vi "HFRR ADV v040.vi"() -> ()   [LabVIEW 2025] (continued)
                    n2687 = local read "FF 2"() -> (→"Frictional Force ( N )" →"Frictional Force ( N )":dbl)
                    n2688 = Build Path(base path=w3261, name or relative path=w3262) -> (appended path=w3257:path)
                    n2689 = flat-sequence {
                      tunnel: w3251 -> [w3317]
                      tunnel: [w3316] -> w3249
                      tunnel: w3248 -> [w3314]
                      tunnel: [w3319] -> w3250
                      tunnel: w3249 -> [w3319]
                      frame #0 {
                        n2690 = call <vilib>:"Mean PtByPt.vi"("x"=w3317, "sample length"="STROKE FILTER", "initialize"=w3314) -> ("mean"=w3316:dbl)  [unwired: 1 in, 1 out]
                      }
                      frame #1 {
                        "STROKE Initialize" <- FALSE ("STROKE Initialize")
                      }
                    }
                    n2691 = local read "COF 2"() -> (w3271:dbl)
                    "Coefficient of Friction" <- w3271
                    "COF 4" <- w3271
                    "Coefficient of Friction" <- w3271
                    n2692 = local read "TEMP"() -> (w3274:dbl)
                    "Temperature ( Deg C )" <- w3274
                    n2693 = local read "Humidity ( %RH )"() -> (w3273:dbl)
                    n2694 = local read "Frequency ( Hz )"() -> (w3280:dbl)
                    n2695 = local read "LVDT STROKE DISPLAY"() -> (w3252:dbl)
                    n2696 = local read "Elapsed time"() -> (w3305:dbl)
                    n2697 = local read "AIR TEMP"() -> (w3278:dbl)
                    n2698 = local read "PID-out"() -> (w3283:dbl)
                    n2699 = local write "Temperature ( Deg C )"(w3274) -> ()
                    n2700 = Number To Fractional String(number=w3252, width (-)=i16 9 ("precision (6)"), precision (6)=i16 6) -> (F-format string=w3298:string)  [unwired: 1 in]
                    n2701 = Number To Fractional String(number=w3278, width (-)=i16 9 ("precision (6)"), precision (6)=i16 3) -> (F-format string=w3297:string)  [unwired: 1 in]
                    n2702 = Number To Fractional String(number=w3274, width (-)=i16 9 ("precision (6)"), precision (6)=i16 3) -> (F-format string=w3294:string)  [unwired: 1 in]
                    n2703 = Number To Fractional String(number=w3273, width (-)=i16 9 ("precision (6)"), precision (6)=i16 3) -> (F-format string=w3291:string)  [unwired: 1 in]
                    n2704 = Number To Fractional String(number=0.0, width (-)=i16 9 ("precision (6)"), precision (6)=i16 3) -> (F-format string=w3288:string)  [unwired: 1 in]
                    n2705 = Number To Fractional String(number=w3283, width (-)=i16 9 ("precision (6)"), precision (6)=i16 3) -> (F-format string=w3284:string)  [unwired: 1 in]
                    n2706 = Number To Fractional String(number=w3280, width (-)=i16 9 ("precision (6)"), precision (6)=i16 3) -> (F-format string=w3279:string)  [unwired: 1 in]
                    n2707 = Number To Fractional String(number=w3271, width (-)=i16 9 ("precision (6)"), precision (6)=i16 6) -> (F-format string=w3306:string)  [unwired: 1 in]
                    n2708 = Number To Fractional String(number=w3305, width (-)=i16 14 ("precision (6)"), precision (6)=i16 3) -> (F-format string=w3307:string)  [unwired: 1 in]
                    n2709 = Bundle("y"=1.02, "LVDT STROKE DISPLAY"=w3252, "y"=0.98) -> (w3272:T31)  [unwired: 1 in]
                    n2710 = Number To Fractional String(number="Ambient Humidity :", width (-)=i16 9 ("precision (6)"), precision (6)=i16 6) -> (F-format string=w3264:string)  [unwired: 1 in]
                    n2711 = local read "RUN"() -> (w3270:bool)
                    n2712 = case shown="True" w3270 {
                      tunnel: w3272 -> [_ w3323]
                      tunnel: w3252 -> [_ w3322]
                      tunnel: w3252 -> [_ w3320]
                      tunnel: w3252 -> [_ w3321]
                      frame False {
                      }
                      frame True {
                        "Stroke ( mm )" <- w3323
                        "Stroke ( mm )" <- w3323
                        "Stroke 4" <- w3322
                        "Stroke 3" <- w3320
                        "Stroke 2" <- w3321
                        "measured_stroke" <- w3320
                      }
                    }
                    n2713 = Concatenate Strings(w3307, w3266, w3306, w3266, w3298, w3266, w3297, w3266, w3294, w3266, w3291, w3266, w3288, w3266, w3284, w3266, w3279, w3266, w3264, "\r") -> (w3304:string)
                    n2714 = call <vilib>:"Write Characters To File.vi"("append to file? (new file:F)"=TRUE, "character string"=w3304, "file path (dialog if empty)"=w3257) -> ()  [unwired: 2 in, 1 out]
                    "refresh flag" <- TRUE ("refresh flag")
                    "LVDT STROKE Actual" <- w3250
                  }
                }
                n2715 = case shown="True" w3172 {
                  tunnel: w3182 -> [_ w3208]
                  tunnel: w3187 -> [_ w3218]
                  tunnel: [0.0 w3214] -> _
                  tunnel: w3181 -> [_ w3213]
                  tunnel: [0.0 w3212] -> _
                  tunnel: w3171 -> [_ w3212]
                  tunnel: w3185 -> [w3201 _]
                  frame False {
                    n2716 = local write "acq timer"(w3201) -> ()
                    n2717 = local write "Test Duration Status"(0.0 ("Test Duration Status")) -> ()
                  }
                  frame True {
                    n2718 = local read "Set Hz"() -> (w3215:dbl)
                    n2719 = local write "Elapsed time"(w3208) -> ()
                    n2720 = local read "test time"() -> (w3207:dbl)
                    n2721 = Multiply(x=w3218, y=w3215) -> (x*y=w3217:dbl)
                    n2722 = case shown="False" w3213 {
                      tunnel: w3217 -> [w3219 _]
                      tunnel: [w3219 1.0] -> w3214
                      frame False {
                        n2723 = local write "Cycles elapsed"(w3219) -> ()
                      }
                      frame True {
                      }
                    }
                    n2724 = Greater?(x=w3208, y=w3207) -> (0:w3216:bool)
                    n2725 = Subtract(x=w3207, y=w3208) -> (x-y=w3206:dbl)
                    n2726 = Multiply(x=w3206, y=60.0) -> (x*y=w3205:dbl)
                    n2727 = local write "Time Remaining"(w3205) -> ()
                    n2728 = local write "Remaining Time"(w3205) -> ()
                    n2729 = case shown="True" w3216 {
                      frame False {
                      }
                      frame True {
                        n2730 = stacked-sequence {
                          frame #0 {
                            w3224 = T19."Enabled" ("Disabled")
                            w3223 = FALSE ("TEST FILE NAM,E SAVED")
                            w3225 = "" ("FILE")
                            w3226 = TRUE ("Visible")
                            n2731 = local write "Humidity"(FALSE ("Humidity")) -> ()
                            n2732 = local write "RUN"(FALSE ("OK Button 2")) -> ()
                            n2733 = local write "Heater Button"(FALSE ("Heater Button")) -> ()
                            n2734 = local write "Auto Start Test"(FALSE ("Auto Start Test")) -> ()
                            n2735 = local write "TestCompFlg"(TRUE ("StpFlg")) -> ()
                            n2736 = local read "Humidity ( %RH )"() -> (→"Rh After":dbl)
                            n2737 = property on="STOP 2" class="Bool (strict)"("Disabled"=u8 0) -> ()  [unwired: 2 in, 2 out]
                            n2738 = local read "EVENT LOG"() -> (w3231:string)
                            n2739 = call "Event Log.vi"("Content"="Test Completed", "EVENT LOG"=w3231) -> ("EVENT LOG"=w3230:string)  [unwired: 8 in, 1 out]
                            n2740 = property on="RUN" class="Bool (strict)"("Visible"=w3226) -> ()  [unwired: 2 in, 2 out]
                            n2741 = property on="Auto Start Test" class="Bool (strict)"("Visible"=w3226) -> ()  [unwired: 2 in, 2 out]
                            n2742 = local write "Batch Ref Num :"(w3225) -> ()
                            n2743 = local write "FILE"(w3225) -> ()
                            n2744 = local write "EVENT LOG"(w3230) -> ()
                            n2745 = local write "TEST FILE NAM,E SAVED"(w3223) -> ()
                            n2746 = local write "Fuel Discription :"(w3225) -> ()
                            n2747 = local write "START TEMP"(w3223) -> ()
                            n2748 = local write "Remarks :"(w3225) -> ()
                            n2749 = local write "Main Dashboard Buttons"(T1."Imaging" ("Main Dashboard Buttons")) -> ()
                            n2750 = local write "Main Tab"(T2."Adv Scar" ("Main Tab")) -> ()
                            n2751 = property on="FRICVALZ 2" class="Bool (strict)"("DisabledEnum"=w3224) -> ()  [unwired: 2 in, 2 out]
                            n2752 = property on="FRICVALZ 3" class="Bool (strict)"("DisabledEnum"=w3224) -> ()  [unwired: 2 in, 2 out]
                            n2753 = property on="FRICVALZ 4" class="Bool (strict)"("DisabledEnum"=w3224) -> ()  [unwired: 2 in, 2 out]
                          }
                          frame #1 {
                            n2754 = Wait (ms)(milliseconds to wait=u32 1500) -> ()  [unwired: 1 out]
                          }
                          frame #2 {
                            n2755 = local write "Due Write"("VC;0") -> ()
                          }
                          frame #3 {
                            n2756 = Wait (ms)(milliseconds to wait=u32 1500) -> ()  [unwired: 1 out]
                          }
                          frame #4 {
                            n2757 = local write "Due Write"("VC;0") -> ()
                          }
                          frame #5 {
                            n2758 = Wait (ms)(milliseconds to wait=u32 1500) -> ()  [unwired: 1 out]
                          }
                          frame #6 {
                            n2759 = local write "Due Write"("ST;0") -> ()
                          }
                          frame #7 {
                            n2760 = local write "measured_stroke"(0.0 ("measured_stroke")) -> ()
                            n2761 = Wait (ms)(milliseconds to wait=u32 1500) -> ()  [unwired: 1 out]
                          }
                          frame #8 {
                            n2762 = local write "Due Write"("HE;0") -> ()
                            n2763 = local write "Humidity 2"(TRUE ("Humidity")) -> ()
                          }
                        }
                      }
                    }
                    n2764 = Divide(x=w3208, y=w3207) -> (x/y=w3211:dbl)
                    n2765 = Multiply(x=w3211, y=100.0) -> (x*y=w3209:dbl)
                    n2766 = local write "Test Duration Status"(w3209) -> ()
                  }
                }
              }
              frame #2 {
                n2767 = case shown="True" "Heater Button" {
                  tunnel: [0.0 ("output") w3346] -> w3324
                  frame False {
                    w3327 = TRUE ("tmpchk")
                    n2768 = local read "TEMP"() -> (w3328:dbl)
                    n2769 = local write "Temp ini"(w3328) -> ()
                    n2770 = local write "Reset 4"(w3327) -> ()
                    n2771 = local write "tmpchk"(w3327) -> ()
                    n2772 = local write "reinit"(TRUE ("reinit")) -> ()
                    n2773 = local write "manual temp log"(TRUE ("manual temp log")) -> ()
                  }
                  frame True {
                    # "Logic to turn off\nthe heater when \ntemp is not rising.\nTime - 60 sec\nDelta t- 5°c"
                    n2774 = local read "Temp ini"() -> (w3335:dbl)
                    n2775 = local read "Auto Start Test"() -> (w3331:bool)
                    n2776 = Less?(x=w3335, y=53.0) -> (x < y?=w3333:bool)
                    n2777 = case shown="False" w3331 {
                      frame False {
                        n2778 = local read "Set Temp"() -> (w3355:dbl)
                        n2779 = local read "TEMP"() -> (w3354:dbl)
                        n2780 = Subtract(x=w3355, y=w3354) -> (x-y=w3353:dbl)
                        n2781 = Absolute Value(x=w3353) -> (abs(x)=w3352:dbl)
                        n2782 = Less?(x=w3352, y=0.5) -> (x < y?=w3350:bool)
                        n2783 = case shown="True" w3350 {
                          tunnel: "manual temp log" -> [_ w3356]
                          frame False {
                          }
                          frame True {
                            n2784 = case shown="True" w3356 {
                              selector: w3356 -> [_ w3357]
                              frame False {
                              }
                              frame True {
                                # "#Event log"
                                n2785 = Not(x=w3357) -> (.not. x?=w3358:bool)
                                n2786 = local write "manual temp log"(w3358) -> ()
                                n2787 = local read "EVENT LOG"() -> (w3361:string)
                                n2788 = call "Event Log.vi"("Content"="Target Temperature reached", "EVENT LOG"=w3361) -> ("EVENT LOG"=w3360:string)  [unwired: 8 in, 1 out]
                                n2789 = local write "EVENT LOG"(w3360) -> ()
                              }
                            }
                          }
                        }
                      }
                      frame True {
                        n2790 = local write "manual temp log"(TRUE ("manual temp log")) -> ()
                      }
                    }
                    n2791 = And(x="tmpchk", y=w3333) -> (x .and. y?=w3336:bool)
                    n2792 = case shown="True" w3336 {
                      frame False {
                      }
                      frame True {
                        n2793 = call "Elapsed Time8"("Time Target (s)"=300.0, "Reset"="Reset 4") -> ("Time has Elapsed"=w3363:bool)  [unwired: 10 in, 7 out]
                        n2794 = flat-sequence {
                          tunnel: w3363 -> [_]
                          frame #0 {
                            n2795 = local write "Reset 4"(FALSE ("Reset 4")) -> ()
                          }
                        }
                        n2796 = case shown="True" w3363 {
                          frame False {
                          }
                          frame True {
                            n2797 = local read "Temp ini"() -> (w3370:dbl)
                            n2798 = Add(x=w3370, y=5.0) -> (x+y=w3368:dbl)
                            n2799 = local read "TEMP"() -> (w3371:dbl)
                            n2800 = Greater?(x=w3371, y=w3368) -> (0:w3369:bool)
                            n2801 = case shown="False" w3369 {
                              frame False {
                                n2802 = local write "Heater Button"(FALSE ("Heater Button")) -> ()
                              }
                              frame True {
                                n2803 = local write "tmpchk"(FALSE ("tmpchk")) -> ()
                              }
                            }
                          }
                        }
                      }
                    }
                    n2804 = local read "Set Temp"() -> (w3344:dbl)
                    n2805 = local read "TEMP"() -> (w3338:dbl)
                    n2806 = call-poly <vilib>:"PID.vi"("reinitialize? (F)"="reinit", "dt (s)"=-1.0, "process variable"=w3338, "setpoint"=w3344) -> ("output"=w3341:dbl)  [unwired: 6 in, 1 out]
                    n2807 = Subtract(x=w3344, y=w3338) -> (x-y=w3345:dbl)
                    n2808 = Add(x=w3344, y=0.5) -> (x+y=w3342:dbl)
                    n2809 = Greater Or Equal?(x=w3338, y=w3342) -> ()  [unwired: 1 out]
                    n2810 = Select(t=0.0, s=FALSE, f=w3341) -> (s? t:f=w3340:dbl)
                    "PID output" <- w3340
                    n2811 = flat-sequence {
                      tunnel: w3340 -> [w3374]
                      tunnel: [w3374] -> w3346
                      frame #0 {
                        n2812 = local write "reinit"(FALSE ("reinit")) -> ()
                      }
                    }
                    n2813 = Bundle(w3345, "output"=w3340, "TEMP"=w3338) -> ()  [unwired: 1 in, 1 out]
                  }
                }
                "PID-out" <- w3324
              }
              frame #3 {
                n2814 = local read "TEMP"() -> (w3376:dbl)
                n2815 = Greater Or Equal?(x=w3376, y="Set Temp 2") -> (x >= y?=w3381:bool)
                n2816 = case shown="True" w3381 {
                  tunnel: [FALSE TRUE] -> w3379
                  frame False {
                  }
                  frame True {
                  }
                }
                "Status 13" <- w3379
                n2817 = And(x=w3379, y="trip1 8") -> (x .and. y?=w3378:bool)
                n2818 = case shown="True" w3378 {
                  frame False {
                    n2819 = local write "Heater Trip Temp"(TRUE ("Heater Trip Temp")) -> ()
                  }
                  frame True {
                    w3384 = FALSE ("OK Button 2")
                    n2820 = case shown="True" "Heater Trip Temp" {
                      selector: "Heater Trip Temp" -> [_ w3386]
                      frame False {
                      }
                      frame True {
                        n2821 = Not(x=w3386) -> (.not. x?=w3385:bool)
                        n2822 = local read "EVENT LOG"() -> (w3389:string)
                        n2823 = local write "Heater Trip Temp"(w3385) -> ()
                        n2824 = call "Event Log.vi"("Content"="Heater Trip", "EVENT LOG"=w3389) -> ("EVENT LOG"=w3388:string)  [unwired: 8 in, 1 out]
                        n2825 = local write "EVENT LOG"(w3388) -> ()
                      }
                    }
                    n2826 = local write "RUN"(w3384) -> ()
                    n2827 = property on="Auto Start Test" class="Bool (strict)"("Value"=w3384) -> ()  [unwired: 2 in, 2 out]
                    n2828 = local write "Heater Button"(w3384) -> ()
                  }
                }
              }
            }
            n2829 = case shown="False" w3095 {
              frame False {
                n2830 = disable-structure shown="Disabled" {
                  frame Disabled {
                    n2831 = stacked-sequence {
                      frame #0 {
                        n2832 = local write "RUN"(FALSE ("OK Button 2")) -> ()
                      }
                      frame #1 {
                      }
                    }
                  }
                  frame Enabled {
                  }
                }
              }
              frame True {
              }
            }
          }
        }
        n2833 = local read "Reset Graph"() -> (w2992:bool)
        n2834 = case shown="True" w2992 {
          selector: w2992 -> [_ w3009]
          frame False {
          }
          frame True {
            w3023 = 0.0 ("X Scale.Range:Maximum")
            n2835 = Not(x=w3009) -> (.not. x?=w3008:bool)
            n2836 = local write "Reset Graph"(w3008) -> ()
            n2837 = property on="Electrical Contact Resistance ( % )" class="WFChart (strict)"("XScale.Maximum"=600.0 ("X Scale.Range:Maximum"), "XScale.Minimum"=0.0 ("X Scale.Range:Minimum"), "YScale.Maximum"=100.0 ("Y Scale.Range:Maximum"), "YScale.Minimum"=0.0 ("Y Scale.Range:Minimum")) -> ()  [unwired: 2 in, 2 out]
            n2838 = property on="Frictional Force ( N )" class="WFChart (strict)"("XScale.Maximum"=600.0 ("X Scale.Range:Maximum"), "XScale.Minimum"=0.0 ("X Scale.Range:Minimum"), "YScale.Maximum"=100.0 ("Y Scale.Range:Maximum"), "YScale.Minimum"=0.0 ("Y Scale.Range:Minimum")) -> ()  [unwired: 2 in, 2 out]
            n2839 = property on="Temperature ( Deg C )" class="WFChart (strict)"("XScale.Maximum"=600.0 ("X Scale.Range:Maximum"), "XScale.Minimum"=0.0 ("X Scale.Range:Minimum"), "YScale.Maximum"=100.0 ("Y Scale.Range:Maximum"), "YScale.Minimum"=0.0 ("Y Scale.Range:Minimum")) -> ()  [unwired: 2 in, 2 out]
            n2840 = property on="Stroke ( mm )" class="WFChart (strict)"("XScale.Maximum"=600.0 ("X Scale.Range:Maximum"), "XScale.Minimum"=0.0 ("X Scale.Range:Minimum"), "YScale.Maximum"=100.0 ("Y Scale.Range:Maximum"), "YScale.Minimum"=0.0 ("Y Scale.Range:Minimum")) -> ()  [unwired: 2 in, 2 out]
            n2841 = property on="Coefficient of Friction" class="WFChart (strict)"("XScale.Maximum"=600.0 ("X Scale.Range:Maximum"), "XScale.Minimum"=0.0 ("X Scale.Range:Minimum"), "YScale.Maximum"=100.0 ("Y Scale.Range:Maximum"), "YScale.Minimum"=0.0 ("Y Scale.Range:Minimum")) -> ()  [unwired: 2 in, 2 out]
            n2842 = property on="Electrical Contact Resistance ( % )" class="WFChart (strict)"("XScale.Minimum"=0.0 ("X Scale.Range:Minimum"), "XScale.Maximum"=600.0 ("X Scale.Range:Maximum"), "YScale.Minimum"=0.0 ("Y Scale.Range:Minimum"), "YScale.Maximum"=100.0 ("Y Scale.Range:Maximum")) -> ()  [unwired: 2 in, 2 out]
            n2843 = property on="Temperature ( Deg C )" class="WFChart (strict)"("XScale.Minimum"=0.0 ("X Scale.Range:Minimum"), "XScale.Maximum"=600.0 ("X Scale.Range:Maximum"), "YScale.Minimum"=0.0 ("Y Scale.Range:Minimum"), "YScale.Maximum"=100.0 ("Y Scale.Range:Maximum")) -> ()  [unwired: 2 in, 2 out]
            n2844 = property on="Coefficient of Friction" class="WFChart (strict)"("XScale.Minimum"=0.0 ("X Scale.Range:Minimum"), "XScale.Maximum"=600.0 ("X Scale.Range:Maximum"), "YScale.Maximum"=1.0 ("X Scale.Range:Minimum"), "YScale.Minimum"=0.0 ("X Scale.Range:Minimum")) -> ()  [unwired: 2 in, 2 out]
            n2845 = property on="Frictional Force ( N )" class="WFChart (strict)"("XScale.Maximum"=600.0 ("X Scale.Range:Maximum"), "XScale.Minimum"=w3023, "YScale.Maximum"=10.0 ("Y Scale.Range:Maximum"), "YScale.Minimum"=w3023) -> ()  [unwired: 2 in, 2 out]
            n2846 = property on="Stroke ( mm )" class="WFChart (strict)"("XScale.Maximum"=600.0 ("X Scale.Range:Maximum"), "XScale.Minimum"=0.0 ("X Scale.Range:Minimum"), "YScale.Maximum"=100.0 ("Y Scale.Range:Maximum"), "YScale.Minimum"=0.0 ("Y Scale.Range:Minimum")) -> ()  [unwired: 2 in, 2 out]
          }
        }
      }
      frame "Compare Files" {
        # "Elapsed time\ncof\nstroke\nAir temp\nTemp\nHumidity"
        n2847 = case shown="True" "RSTV1 2" {
          frame False {
          }
          frame True {
            n2848 = property on="Humidity ( %RH )" class="XYGraph (strict)"("Y Scale.Display Format:Precision"=u8 0 ("Y Scale.Format & Precision:Precision")) -> ()  [unwired: 2 in, 2 out]
            n2849 = property on="Humidity ( %RH )" class="XYGraph (strict)"("X Scale.Range:Minimum"=0.0, "X Scale.Range:Maximum"=75.0, "Y Scale.Range:Minimum"=48.0, "Y Scale.Range:Maximum"=58.0) -> ()  [unwired: 2 in, 2 out]
          }
        }
        n2850 = case shown="True" "RST CP 2" {
          frame False {
          }
          frame True {
            n2851 = property on="XY Graph 13" class="XYGraph (strict)"("Y Scale.Display Format:Precision"=u8 0 ("Y Scale.Format & Precision:Precision")) -> ()  [unwired: 2 in, 2 out]
            n2852 = property on="XY Graph 13" class="XYGraph (strict)"("X Scale.Range:Minimum"=0.0, "X Scale.Range:Maximum"=75.0, "Y Scale.Range:Minimum"=0.0, "Y Scale.Range:Maximum"=100.0) -> ()  [unwired: 2 in, 2 out]
          }
        }
        n2853 = case shown="True" "RST CP" {
          frame False {
          }
          frame True {
            n2854 = property on="Sample Temperature ( °C )" class="XYGraph (strict)"("Y Scale.Display Format:Precision"=u8 2 ("Y Scale.Format & Precision:Precision")) -> ()  [unwired: 2 in, 2 out]
            n2855 = property on="Sample Temperature ( °C )" class="XYGraph (strict)"("X Scale.Range:Minimum"=0.0, "X Scale.Range:Maximum"=75.0, "Y Scale.Range:Minimum"=58.0, "Y Scale.Range:Maximum"=62.0) -> ()  [unwired: 2 in, 2 out]
          }
        }
        n2856 = case shown="True" "RSTV1 3" {
          frame False {
          }
          frame True {
            n2857 = property on="Air Temperature  ( °C )" class="XYGraph (strict)"("Y Scale.Display Format:Precision"=u8 2 ("Y Scale.Format & Precision:Precision")) -> ()  [unwired: 2 in, 2 out]
            n2858 = property on="Air Temperature  ( °C )" class="XYGraph (strict)"("X Scale.Range:Minimum"=0.0 ("Y Scale.Range:Minimum"), "X Scale.Range:Maximum"=75.0 ("Y Scale.Range:Maximum"), "Y Scale.Range:Minimum"=20.0 ("X Scale.Range:Minimum"), "Y Scale.Range:Maximum"=26.0 ("X Scale.Range:Maximum")) -> ()  [unwired: 2 in, 2 out]
          }
        }
        n2859 = case shown="True" "RSTV1 4" {
          frame False {
          }
          frame True {
            n2860 = property on="Stroke ( mm )" class="XYGraph (strict)"("Y Scale.Display Format:Precision"=u8 2 ("Y Scale.Format & Precision:Precision")) -> ()  [unwired: 2 in, 2 out]
            n2861 = property on="Stroke ( mm )" class="XYGraph (strict)"("X Scale.Range:Minimum"=0.0 ("Y Scale.Range:Maximum"), "X Scale.Range:Maximum"=75.0 ("X Scale.Range:Minimum"), "Y Scale.Range:Minimum"=0.98, "Y Scale.Range:Maximum"=1.02) -> ()  [unwired: 2 in, 2 out]
          }
        }
        n2862 = case shown="True" "rstv2" {
          frame False {
          }
          frame True {
            n2863 = property on="Coefficient Of Friction" class="XYGraph (strict)"("Y Scale.Display Format:Precision"=u8 3 ("Y Scale.Format & Precision:Precision")) -> ()  [unwired: 2 in, 2 out]
            n2864 = property on="Coefficient Of Friction" class="XYGraph (strict)"("X Scale.Range:Minimum"=0.0 ("Y Scale.Range:Maximum"), "X Scale.Range:Maximum"=75.0, "Y Scale.Range:Minimum"=0.0, "Y Scale.Range:Maximum"=1.0 ("X Scale.Range:Minimum")) -> ()  [unwired: 2 in, 2 out]
          }
        }
        n2865 = case shown="True" "RST CP 3" {
          frame False {
          }
          frame True {
            n2866 = property on="Air Temp ( °C ) vs Humidity ( % RH )" class="XYGraph (strict)"("X Scale.Range:Minimum"=18.0, "X Scale.Range:Maximum"=28.0 ("X Scale.Range:Minimum"), "Y Scale.Range:Minimum"=30.0 ("X Scale.Range:Minimum"), "Y Scale.Range:Maximum"=70.0 ("X Scale.Range:Minimum")) -> ()  [unwired: 2 in, 2 out]
          }
        }
        n2867 = case shown="True" "OPEN 1" {
          frame False {
          }
          frame True {
            (unwired) 0  # existing file
            w3665 = "Choose a datalog file to open"  # prompt
            n2868 = local write "OPEN 1"(FALSE ("OPEN 1")) -> ()
            n2869 = String To Path(string="C:\\LAB-IQ\\Data\\") -> (path=w3650:path)
            n2870 = File Dialog(6:"*.dgf" ("pattern"), 7:w3665, 11:w3650) -> (0:w3648:errorcluster, 3:w3656:path)  [unwired: 4 in, 2 out]
            n2871 = Unbundle(w3648) -> ()  [unwired: 3 out]
            n2872 = Strip Path(path=w3656) -> (name=w3655:string)  [unwired: 1 out]
            n2873 = Path To String(path=w3656) -> (string=w3651:string)
            "string1" <- w3651
            n2874 = Match Pattern(string=w3655, regular expression=".dgf") -> (before substring=→"String Control":string)  [unwired: 1 in, 3 out]
            n2875 = Match Pattern(string=w3651, regular expression=".dgf" ("substring (\"\")")) -> (before substring=w3661:string)  [unwired: 1 in, 3 out]
            n2876 = Concatenate Strings(w3661, ".duf" ("Substring")) -> (w3657:string)
            n2877 = String To Path(string=w3657) -> (path=w3662:path)
            n2878 = call <vilib>:"Read Characters From File.vi"("file path (dialog if empty)"=w3662, "start of read offset (chars.:0)"=60 ("start of read offset (chars.: 0)")) -> ("character string"=→"String Control 2":string)  [unwired: 4 in, 3 out]
          }
        }
        n2879 = case shown="True" "OPEN 2" {
          frame False {
          }
          frame True {
            (unwired) 0  # existing file
            w3683 = "Choose a datalog file to open"  # prompt
            n2880 = local write "OPEN 2"(FALSE ("OPEN 1")) -> ()
            n2881 = String To Path(string="C:\\LAB-IQ\\Data\\") -> (path=w3668:path)
            n2882 = File Dialog(6:"*.dgf" ("pattern"), 7:w3683, 11:w3668) -> (0:w3666:errorcluster, 3:w3674:path)  [unwired: 4 in, 2 out]
            n2883 = Unbundle(w3666) -> ()  [unwired: 3 out]
            n2884 = Strip Path(path=w3674) -> (name=w3672:string)  [unwired: 1 out]
            n2885 = Path To String(path=w3674) -> (string=w3669:string)
            "string1 2" <- w3669
            n2886 = Match Pattern(string=w3672, regular expression=".dgf") -> (before substring=→"String Control 3":string)  [unwired: 1 in, 3 out]
            n2887 = Match Pattern(string=w3669, regular expression=".dgf" ("substring (\"\")")) -> (before substring=w3680:string)  [unwired: 1 in, 3 out]
            n2888 = Concatenate Strings(w3680, ".duf" ("Substring")) -> (w3677:string)
            n2889 = String To Path(string=w3677) -> (path=w3675:path)
            n2890 = call <vilib>:"Read Characters From File.vi"("file path (dialog if empty)"=w3675, "start of read offset (chars.:0)"=60 ("start of read offset (chars.: 0)")) -> ("character string"=→"String Control 4":string)  [unwired: 4 in, 3 out]
          }
        }
        n2891 = case shown="True" "OPEN 3" {
          frame False {
          }
          frame True {
            (unwired) 0  # existing file
            w3701 = "Choose a datalog file to open"  # prompt
            n2892 = local write "OPEN 3"(FALSE ("OPEN 1")) -> ()
            n2893 = String To Path(string="C:\\LAB-IQ\\Data\\") -> (path=w3686:path)
            n2894 = File Dialog(6:"*.dgf" ("pattern"), 7:w3701, 11:w3686) -> (0:w3684:errorcluster, 3:w3692:path)  [unwired: 4 in, 2 out]
            n2895 = Unbundle(w3684) -> ()  [unwired: 3 out]
            n2896 = Strip Path(path=w3692) -> (name=w3690:string)  [unwired: 1 out]
            n2897 = Path To String(path=w3692) -> (string=w3687:string)
            "string1 3" <- w3687
            n2898 = Match Pattern(string=w3690, regular expression=".dgf") -> (before substring=→"String Control 5":string)  [unwired: 1 in, 3 out]
            n2899 = Match Pattern(string=w3687, regular expression=".dgf" ("substring (\"\")")) -> (before substring=w3697:string)  [unwired: 1 in, 3 out]
            n2900 = Concatenate Strings(w3697, ".duf" ("Substring")) -> (w3694:string)
            n2901 = String To Path(string=w3694) -> (path=w3698:path)
            n2902 = call <vilib>:"Read Characters From File.vi"("file path (dialog if empty)"=w3698, "start of read offset (chars.:0)"=60 ("start of read offset (chars.: 0)")) -> ("character string"=→"String Control 6":string)  [unwired: 4 in, 3 out]
          }
        }
        n2903 = case shown="True" "OPEN 4" {
          frame False {
          }
          frame True {
            (unwired) 0  # existing file
            w3719 = "Choose a datalog file to open"  # prompt
            n2904 = local write "OPEN 4"(FALSE ("OPEN 1")) -> ()
            n2905 = String To Path(string="C:\\LAB-IQ\\Data\\") -> (path=w3704:path)
            n2906 = File Dialog(6:"*.dgf" ("pattern"), 7:w3719, 11:w3704) -> (0:w3702:errorcluster, 3:w3710:path)  [unwired: 4 in, 2 out]
            n2907 = Unbundle(w3702) -> ()  [unwired: 3 out]
            n2908 = Strip Path(path=w3710) -> (name=w3708:string)  [unwired: 1 out]
            n2909 = Path To String(path=w3710) -> (string=w3705:string)
            "string1 4" <- w3705
            n2910 = Match Pattern(string=w3708, regular expression=".dgf") -> (before substring=→"String Control 7":string)  [unwired: 1 in, 3 out]
            n2911 = Match Pattern(string=w3705, regular expression=".dgf" ("substring (\"\")")) -> (before substring=w3715:string)  [unwired: 1 in, 3 out]
            n2912 = Concatenate Strings(w3715, ".duf" ("Substring")) -> (w3712:string)
            n2913 = String To Path(string=w3712) -> (path=w3716:path)
            n2914 = call <vilib>:"Read Characters From File.vi"("file path (dialog if empty)"=w3716, "start of read offset (chars.:0)"=60 ("start of read offset (chars.: 0)")) -> ("character string"=→"String Control 8":string)  [unwired: 4 in, 3 out]
          }
        }
      }
      frame "About" {
        # "Elapsed time\ncof\nstroke\nmean pos\nTemp\nHumidity"
        n2915 = disable-structure shown="Disabled" {
          frame Disabled {
            n2916 = case shown="True" "Export" {
              frame False {
              }
              frame True {
                w3741 = "                                      " ("string")
                w3743 = "\r"
                (unwired) i16 6 ("width (-)")
                w3820 = "\r"
                w3752 = "\r"
                n2917 = local write "Export"(FALSE ("Export")) -> ()
                n2918 = local read "String 29"() -> (w3789:string)
                n2919 = local read "String 34"() -> (w3777:string)
                n2920 = local read "String 35"() -> (w3772:string)
                n2921 = local read "String 37"() -> (w3768:string)
                n2922 = local read "String 36"() -> (w3765:string)
                n2923 = local read "String 38"() -> (w3762:string)
                n2924 = local read "String 39"() -> (w3759:string)
                n2925 = Match Pattern(string=w3789, regular expression=".dwm") -> (before substring=w3785:string)  [unwired: 1 in, 3 out]
                "before substring" <- w3785
                n2926 = local read "S 38"() -> (w3780:string)
                n2927 = local read "S 39"() -> (w3773:string)
                n2928 = local read "Temperature before test 2"() -> (w3809:dbl)
                n2929 = local read "Temperature after test 2"() -> (w3814:dbl)
                n2930 = local read "Humidity before test 2"() -> (w3795:dbl)
                n2931 = local read "Humidity after test 2"() -> (w3810:dbl)
                n2932 = local read "MWSD 2"() -> (w3806:dbl)
                n2933 = local read "WS1.4 2"() -> (w3822:dbl)
                n2934 = local read "HCF 2"() -> (w3818:dbl)
                n2935 = local read "AVP 2"() -> (w3807:dbl)
                n2936 = Concatenate Strings("1," ("string"), w3780) -> (w3779:string)
                n2937 = Concatenate Strings("2," ("string"), w3777) -> (w3776:string)
                n2938 = Concatenate Strings("3," ("string"), w3773) -> (w3775:string)
                n2939 = Concatenate Strings("4," ("string"), w3772) -> (w3771:string)
                n2940 = Concatenate Strings("5," ("string"), w3768) -> (w3769:string)
                n2941 = Concatenate Strings("6," ("string"), w3765) -> (w3766:string)
                n2942 = Concatenate Strings("7," ("string"), w3762) -> (w3763:string)
                n2943 = Concatenate Strings("8," ("string"), w3759) -> (w3760:string)
                n2944 = local read "Sample ID"() -> (w3827:string)
                n2945 = case shown="\"xlx\"" "Select File Type" {
                  tunnel: w3785 -> [w3830 w3832 w3834]
                  tunnel: [w3828 w3833 w3835] -> w3784
                  frame "xlx" {
                    n2946 = Concatenate Strings(w3830, ".xls" ("string")) -> (w3828:string)
                  }
                  frame "csv" {
                    n2947 = Concatenate Strings(w3832, ".csv" ("string")) -> (w3833:string)
                  }
                  frame "txt" {
                    n2948 = Concatenate Strings(w3834, ".txt" ("string")) -> (w3835:string)
                  }
                }
                n2949 = local read "Test Date"() -> (w3826:string)
                n2950 = local read "String 45"() -> (w3740:string)
                n2951 = local read "String 31"() -> (w3825:string)
                n2952 = local read "String 32"() -> (w3824:string)
                n2953 = local read "TITTLE"() -> (w3748:string)
                n2954 = Number To Fractional String(number=w3795, width (-)=i16 6, precision (6)=i16 2) -> (F-format string=w3794:string)  [unwired: 1 in]
                n2955 = Number To Fractional String(number=w3809, width (-)=i16 6, precision (6)=i16 2) -> (F-format string=w3815:string)  [unwired: 1 in]
                n2956 = Number To Fractional String(number=w3810, width (-)=i16 6, precision (6)=i16 2) -> (F-format string=w3808:string)  [unwired: 1 in]
                n2957 = Number To Fractional String(number=w3814, width (-)=i16 6, precision (6)=i16 2) -> (F-format string=w3813:string)  [unwired: 1 in]
                n2958 = Number To Fractional String(number=w3806, width (-)=i16 6, precision (6)=i16 2) -> (F-format string=w3804:string)  [unwired: 1 in]
                n2959 = Number To Fractional String(number=w3807, width (-)=i16 6, precision (6)=i16 2) -> (F-format string=w3805:string)  [unwired: 1 in]
                n2960 = Number To Fractional String(number=w3818, width (-)=i16 6, precision (6)=i16 2) -> (F-format string=w3819:string)  [unwired: 1 in]
                n2961 = Number To Fractional String(number=w3822, precision (6)=i16 2) -> (F-format string=w3823:string)  [unwired: 2 in]
                n2962 = local read "s.NO"() -> (w3742:string)
                n2963 = Concatenate Strings("=" ("string"), w3748) -> (w3747:string)
                n2964 = Concatenate Strings("S.No," ("string"), "                                       Parameters" ("string")) -> (w3753:string)
                n2965 = Concatenate Strings(w3820, w3779, w3794, w3820, w3776, w3815, w3820, w3775, w3808, w3820, w3771, w3813, w3820, w3769, w3804, w3820, w3766, w3805, w3820, w3763, w3819, w3820, w3760, w3823) -> (w3782:string)
                n2966 = Concatenate Strings(w3752, "," ("string"), w3740, w3742, w3741, w3824, w3827, w3741, w3825, w3826, w3752) -> (w3750:string)
                n2967 = local read "Tested by"() -> (w3756:string)
                n2968 = local read "String 33"() -> (w3757:string)
                n2969 = Concatenate Strings("," ("string"), "                                                                             " ("string")) -> (w3745:string)
                n2970 = Concatenate Strings(w3747, w3743, w3750, w3743, w3753, w3782, w3743, w3745, w3757, w3756) -> (→"export":string)
                n2971 = String To Path(string=w3784) -> (path=w3791:path)
                n2972 = local read "export"() -> (w3786:string)
                n2973 = call <vilib>:"Write Characters To File.vi"("append to file? (new file:F)"=FALSE, "character string"=w3786, "file path (dialog if empty)"=w3791) -> ()  [unwired: 2 in, 1 out]
              }
            }
          }
          frame Enabled {
          }
        }
        n2974 = case shown="True" "OK Button 17" {
          frame False {
          }
          frame True {
            (unwired) 0  # existing file
            w4044 = "Choose a datalog file to open"  # prompt
            n2975 = local write "OK Button 17"(FALSE ("OK Button 17")) -> ()
            n2976 = local read "String"() -> (w4039:string)
            n2977 = String To Path(string=w4039) -> (path=w4040:path)
            n2978 = File Dialog(6:"*.duf" ("pattern"), 7:w4044, 11:w4040) -> (0:w4031:errorcluster, 3:w4050:path)  [unwired: 4 in, 2 out]
            n2979 = Unbundle(w4031) -> ()  [unwired: 3 out]
            n2980 = Open/Create/Replace File "Open File"(file path (use dialog)=w4050) -> (refnum out=w4042:refnum<file>)  [unwired: 5 in, 2 out]
            n2981 = Strip Path(path=w4050) -> (name=w4048:string)  [unwired: 1 out]
            n2982 = Path To String(path=w4050) -> (string=w4033:string)
            n2983 = while {
              tunnel: w4042 -> [w4054]
              i -> [w4051]
              stop <- w4052 continue-if-true
              (unwired) TRUE ("line mode (F)")
              n2984 = Read from Text File "Read File"(file (use dialog)=w4054) -> (text=w4053:string)  [unwired: 3 in, 3 out]
              n2985 = local write "Numeric 16"(w4051) -> ()
              n2986 = String Length(string=w4053) -> (length=w4056:i32)
              n2987 = Greater?(x=w4056, y=1) -> (0:w4052:bool)
            }
            n2988 = local write "String 29"(w4033) -> ()
            n2989 = Search and Replace String(input string=w4033, search string=".duf", replace string=".dgf" ("replace string (\"\")")) -> (result string=→"String Indicator 4":string)  [unwired: 5 in, 3 out]
            n2990 = Match Pattern(string=w4048, regular expression=".dwm") -> (before substring=w4032:string)  [unwired: 1 in, 3 out]
            "String Indicator" <- w4032
            n2991 = Match Pattern(string=w4033, regular expression=".dwm" ("substring (\"\")")) -> (before substring=w4034:string)  [unwired: 1 in, 3 out]
            "String Indicator 3" <- w4034
            n2992 = local write "TITTLE 2"(w4032) -> ()
            n2993 = String To Path(string=w4034) -> (path=w4041:path)
            "path" <- w4041
            n2994 = call <vilib>:"Read Characters From File.vi"("file path (dialog if empty)"=w4041, "start of read offset (chars.:0)"=60 ("start of read offset (chars.: 0)")) -> ("character string"=→"String Indicator 2":string)  [unwired: 4 in, 3 out]
          }
        }
        n2995 = call <vilib>:"Query Available Printers.vi"() -> ("system configured printers"=w3733:string[])  [unwired: 9 in, 2 out]
        "System Configured Printers 2" <- w3733
        n2996 = local read "OK Button 16"() -> (w3730:bool)
        n2997 = case shown="True" "OK Button 16" {
          frame False {
          }
          frame True {
            n2998 = stacked-sequence {
              frame #0 {
                n2999 = local read "Numeric 16"() -> (w4058:i32)
                n3000 = local write "Numeric 10"(w4058) -> ()
              }
              frame #1 {
                n3001 = local read "String 29"() -> (w4061:string)
                n3002 = String To Path(string=w4061) -> (path=w4060:path)
                n3003 = Open/Create/Replace File "Open File"(file path (use dialog)=w4060) -> (refnum out=w4062:refnum<file>)  [unwired: 5 in, 2 out]
                n3004 = for {
                  N: 16 -> [_]
                  tunnel: w4062 -> [w4069]
                  i -> [w4065]
                  (unwired) TRUE ("line mode (F)")
                  n3005 = Read from Text File "Read File"(file (use dialog)=w4069) -> (text=w4063:string)  [unwired: 3 in, 3 out]
                  n3006 = Match Pattern(string=w4063, regular expression="(") -> (after substring=w4068:string)  [unwired: 1 in, 3 out]
                  n3007 = Match Pattern(string=w4068, regular expression=")") -> (before substring=w4064:string)  [unwired: 1 in, 3 out]
                  n3008 = case shown="1" w4065 {
                    tunnel: w4064 -> [w4070 w4071 _ _ w4072 w4073 w4074 w4076 w4078 w4080 w4082 w4084 w4086 w4088 _]
                    tunnel: w4063 -> [_ _ _ _ _ _ _ _ _ _ _ _ _ _ _]
                    frame 0 {
                      "TITTLE" <- w4070
                    }
                    frame 1 {
                      "Sample ID" <- w4071
                    }
                    frame 2 {
                    }
                    frame 3 {
                    }
                    frame 4 {
                      "Test Date" <- w4072
                    }
                    frame 5 {
                      "Tested by" <- w4073
                    }
                    frame 6 {
                      n3009 = Fract/Exp String To Number(string=w4074) -> (number=→"Humidity before test 2":dbl)  [unwired: 3 in, 1 out]
                    }
                    frame 7 {
                      n3010 = Fract/Exp String To Number(string=w4076) -> (number=→"Temperature before test 2":dbl)  [unwired: 3 in, 1 out]
                    }
                    frame 8 {
                      n3011 = Fract/Exp String To Number(string=w4078) -> (number=→"Humidity after test 2":dbl)  [unwired: 3 in, 1 out]
                    }
                    frame 9 {
                      n3012 = Fract/Exp String To Number(string=w4080) -> (number=→"Temperature after test 2":dbl)  [unwired: 3 in, 1 out]
                    }
                    frame 10 {
                      n3013 = Fract/Exp String To Number(string=w4082) -> (number=→"MWSD 2":dbl)  [unwired: 3 in, 1 out]
                    }
                    frame 11 {
                      n3014 = Fract/Exp String To Number(string=w4084) -> (number=→"AVP 2":dbl)  [unwired: 3 in, 1 out]
                    }
                    frame 12 {
                      n3015 = Fract/Exp String To Number(string=w4086) -> (number=→"HCF 2":dbl)  [unwired: 3 in, 1 out]
                    }
                    frame 13 {
                      n3016 = Fract/Exp String To Number(string=w4088) -> (number=→"WS1.4 2":dbl)  [unwired: 3 in, 1 out]
                    }
                    frame 14, Default {
                    }
                  }
                }
              }
              frame #2 {
              }
            }
            n3017 = local write "OK Button 16"(FALSE ("OK Button 13")) -> ()
          }
        }
        n3018 = Index Array(array=w3733, index="Select Printer 3") -> (element=w3735:string)
        "Selected Printer" <- w3735
        n3019 = case shown="True" w3730 {
          frame False {
          }
          frame True {
            n3020 = flat-sequence {
              frame #0 {
              }
              frame #1 {
                n3021 = Wait (ms)(milliseconds to wait=u32 100) -> ()  [unwired: 1 out]
              }
              frame #2 {
                n3022 = local write "OK Button 16"(FALSE ("Print 3")) -> ()
              }
            }
          }
        }
        n3023 = case shown="True" "Print" {
          tunnel: w3735 -> [_ w4027]
          frame False {
          }
          frame True {
            (unwired) i16 6 ("width (-)")
            (unwired) "TESTED BY : "
            (unwired) "TESTED DATE :"
            (unwired) "SAMPLE ID : "
            (unwired) "SAMPLE DESIGN : "
            w3985 = "\r"
            w4002 = "\r"
            # "add image"
            n3024 = local read "Sample ID"() -> (w3975:string)
            n3025 = local read "Tested by"() -> (w3978:string)
            n3026 = local read "String 34"() -> (w3965:string)
            n3027 = local read "String 45"() -> (w3945:string)
            n3028 = local read "String 35"() -> (w3960:string)
            n3029 = local read "String 37"() -> (w3958:string)
            n3030 = local read "String 32"() -> (w3980:string)
            n3031 = local read "String 36"() -> (w3955:string)
            n3032 = local read "String 31"() -> (w3979:string)
            n3033 = local read "Test Date"() -> (w3976:string)
            n3034 = local read "String 33"() -> (w3981:string)
            n3035 = local read "String 38"() -> (w3951:string)
            n3036 = local read "String 39"() -> (w3948:string)
            n3037 = local write "Print"(FALSE ("Print FF")) -> ()
            n3038 = local read "S 39"() -> (w3963:string)
            n3039 = local read "S 38"() -> (w3970:string)
            n3040 = local read "Temperature before test 2"() -> (w4001:dbl)
            n3041 = local read "Temperature after test 2"() -> (w3991:dbl)
            n3042 = local read "Humidity before test 2"() -> (w4016:dbl)
            n3043 = local read "Humidity after test 2"() -> (w4000:dbl)
            n3044 = local read "MWSD 2"() -> (w4005:dbl)
            n3045 = local read "WS1.4 2"() -> (w3983:dbl)
            n3046 = Concatenate Strings("2)" ("string"), w3965) -> (w3966:string)
            n3047 = Concatenate Strings("3)" ("string"), w3963) -> (w3964:string)
            n3048 = Concatenate Strings("1)" ("string"), w3970) -> (w3969:string)
            n3049 = Concatenate Strings("4)" ("string"), w3960) -> (w3961:string)
            n3050 = Concatenate Strings("5)" ("string"), w3958) -> (w3957:string)
            n3051 = Concatenate Strings("6)" ("string"), w3955) -> (w3954:string)
            n3052 = Concatenate Strings("7)" ("string"), w3951) -> (w3952:string)
            n3053 = Concatenate Strings("8)" ("string"), w3948) -> (w3949:string)
            n3054 = local read "HCF 2"() -> (w3987:dbl)
            n3055 = local read "AVP 2"() -> (w4004:dbl)
            n3056 = local read "s.NO"() -> (w3946:string)
            n3057 = call <vilib>:"New Report.vi"("report type"=enum16{"Standard Report", "HTML"}."Standard Report") -> ("report out"=w4025:refnum<class "NI_report.lvclass">, "error out"=w4024:errorcluster)  [unwired: 13 in]
            n3058 = local read "TITTLE"() -> (w3977:string)
            n3059 = Concatenate Strings(w4002, w3945, w3946, w4002, w3980, w3975, w4002, w3979, w3976, w4002, w3981, w3978, w4002) -> (w3995:string)
            "test by" <- w3995
            n3060 = Number To Fractional String(number=w4001, width (-)=i16 6, precision (6)=i16 2) -> (F-format string=w3990:string)  [unwired: 1 in]
            n3061 = Number To Fractional String(number=w4000, width (-)=i16 6, precision (6)=i16 2) -> (F-format string=w4003:string)  [unwired: 1 in]
            n3062 = Number To Fractional String(number=w4016, width (-)=i16 6, precision (6)=i16 2) -> (F-format string=w4021:string)  [unwired: 1 in]
            n3063 = Number To Fractional String(number=w4005, width (-)=i16 6, precision (6)=i16 2) -> (F-format string=w4007:string)  [unwired: 1 in]
            n3064 = Number To Fractional String(number=w3991, width (-)=i16 6, precision (6)=i16 2) -> (F-format string=w3992:string)  [unwired: 1 in]
            n3065 = Number To Fractional String(number=w4004, width (-)=i16 6, precision (6)=i16 2) -> (F-format string=w4006:string)  [unwired: 1 in]
            n3066 = Number To Fractional String(number=w3987, width (-)=i16 6, precision (6)=i16 2) -> (F-format string=w3986:string)  [unwired: 1 in]
            n3067 = Number To Fractional String(number=w3983, precision (6)=i16 2) -> (F-format string=w3982:string)  [unwired: 2 in]
            n3068 = call-dynamic "Set Report Header Text.vi"("report in"=w4025, "center header text"=w3977, "error in (no error)"=w4024) -> ("report out"=w3996:refnum<class "NI_report.lvclass">, "error out"=w3997:errorcluster)  [unwired: 11 in]
            n3069 = Concatenate Strings(w3985, w3969, w4021, w3985, w3966, w3990, w3985, w3964, w4003, w3985, w3961, w3992, w3985, w3957, w4007, w3985, w3954, w4006, w3985, w3952, w3986, w3985, w3949, w3982) -> (w3973:string)
            "export 2" <- w3973
            n3070 = call-poly <vilib>:"Append Report Text.vi"("report in"=w3996, "text"=w3995, "error in (no error)"=w3997) -> ("report out"=w3999:refnum<class "NI_report.lvclass">, "error out"=w3998:errorcluster)  [unwired: 9 in, 2 out]
            n3071 = local read "test by"() -> (w3972:string)
            n3072 = local read "TITTLE"() -> (w3974:string)
            n3073 = call-poly <vilib>:"Append Report Text.vi"("report in"=w3999, "error in (no error)"=w3998) -> ("report out"=w4020:refnum<class "NI_report.lvclass">, "error out"=w4018:errorcluster)  [unwired: 10 in, 2 out]
            n3074 = Concatenate Strings(w3974, w3973, w3972) -> (→"output":string)
            n3075 = call-poly <vilib>:"Append Report Text.vi"("report in"=w4020, "text"=w3973, "error in (no error)"=w4018) -> ("report out"=w4019:refnum<class "NI_report.lvclass">, "error out"=w4017:errorcluster)  [unwired: 9 in, 2 out]
            n3076 = call-dynamic "Print Report.vi"("report in"=w4019, "printer name (default)"=w4027, "error in (no error)"=w4017) -> ("report out"=w4029:refnum<class "NI_report.lvclass">, "error out"=w4030:errorcluster)  [unwired: 11 in]
            n3077 = call-dynamic "Dispose Report.vi"("report in"=w4029, "error in (no error)"=w4030) -> ()  [unwired: 13 in, 1 out]
          }
        }
        n3078 = case shown="True" "Print 2" {
          frame False {
          }
          frame True {
            n3079 = flat-sequence {
              frame #0 {
                n3080 = local read "s.NO"() -> (→"s.NO 2":string)
                n3081 = Wait (ms)(milliseconds to wait=u32 20) -> ()  [unwired: 1 out]
                n3082 = local read "Sample ID  3"() -> (→"Sample ID  6":string)
                n3083 = local read "Sample ID  4"() -> (→"Sample ID  7":string)
                n3084 = local read "Sample ID"() -> (→"Sample ID  2":string)
                n3085 = local read "Tested by"() -> (→"Tested by 2":string)
                n3086 = local read "Test Date"() -> (→"Test Date 2":string)
                n3087 = local read "Humidity after test 3"() -> (→"Humidity after test 4":dbl)
                n3088 = local read "Ref A Test Date :"() -> (→"TITTLE 4":string)
                n3089 = local read "Temperature before test 3"() -> (w3852:dbl)
                n3090 = local read "Temperature before test 3"() -> (→"Temperature after test 5":dbl)
                n3091 = local read "Temperature after test 3"() -> (→"Temperature after test 4":dbl)
                n3092 = local read "Humidity before test 3"() -> (→"Humidity before test 4":dbl)
                n3093 = local write "Temperature before test 3"(w3852) -> ()
                n3094 = local read "image data"() -> (w3843:T16)
                n3095 = String To Path(string="C:\\LAB-IQ\\im\\Temp_resized.jpg") -> (path=w3844:path)
                "path 2" <- w3844
                n3096 = call <vilib>:"Write JPEG File.vi"("image data"=w3843, "path to JPEG file"=w3844) -> ()  [unwired: 8 in, 2 out]
                "Ref A Test Date :" <- "Ref A Test Date :"
                "Ref B Test Date :" <- "Ref B Test Date :"
                "Ref B Scar Value :" <- "Ref B Scar Value :"
                "Ref A Scar Value :" <- "Ref A Scar Value :"
              }
              frame #1 {
                (unwired) HTML_Report_Image_Alignment."MIDDLE" ("alignment (default)")
                w3880 = u16 0 items=["portrait", "landscape"] ("orientation (portrait)")
                (unwired) HTML_Report_Image_Alignment."ABSMIDDLE" ("alignment (default)")
                (unwired) "TESTED BY : "
                (unwired) "TESTED DATE :"
                (unwired) "SAMPLE ID : "
                (unwired) "SAMPLE DESIGN : "
                w3913 = "\r"
                # "add image"
                n3097 = Wait (ms)(milliseconds to wait=u32 20) -> ()  [unwired: 1 out]
                n3098 = local read "Sample ID  2"() -> (w3906:string)
                n3099 = local read "Wear Scar X"() -> (w3878:dbl)
                "Length ( microns ) 2" <- w3878
                n3100 = local read "Wear Scar Y"() -> (w3877:dbl)
                "Wear Scar Y ( microns ) :" <- w3877
                n3101 = local read "Test Date 2"() -> (w3907:string)
                n3102 = local read "Tested by 2"() -> (w3908:string)
                n3103 = local read "String 46"() -> (w3904:string)
                n3104 = local read "String 48"() -> (w3910:string)
                n3105 = local read "String 47"() -> (w3909:string)
                n3106 = local read "String 49"() -> (w3911:string)
                n3107 = local read "String 10"() -> (w3864:string)
                n3108 = local read "s.NO 2"() -> (w3905:string)
                n3109 = Add(x=w3878, y=w3877) -> (x+y=w3876:dbl)
                n3110 = call <vilib>:"New Report.vi"("report type"=enum16{"Standard Report", "HTML"}."HTML") -> ("report out"=w3884:refnum<class "NI_report.lvclass">, "error out"=w3882:errorcluster)  [unwired: 13 in]
                n3111 = Concatenate Strings(w3913, w3904, w3905, w3913, w3910, w3906, w3913, w3909, w3907, w3913, w3911, w3908, w3913) -> (→"test by 2":string)
                n3112 = Concatenate Strings("C:\\LAB-IQ\\Data\\" ("string"), w3864, ".jpg" ("string")) -> ()  [unwired: 1 out]
                n3113 = Divide(x=w3876, y=2.0) -> (x/y=→"Mean Wear ( microns) :":dbl)
                n3114 = call-dynamic "Set Report Orientation.vi"("report in"=w3884, "orientation (portrait)"=w3880, "error in (no error)"=w3882) -> ("report out"=w3883:refnum<class "NI_report.lvclass">, "error out"=w3881:errorcluster)  [unwired: 11 in]
                n3115 = for {
                  N: 5 -> [_]
                  tunnel: w3883 -> [w3934]
                  tunnel: [w3933] -> w3862
                  tunnel: w3881 -> [w3932]
                  tunnel: [w3931] -> w3861
                  n3116 = call-dynamic "Set Report Tab Width.vi"("report in"=w3934, "error in (no error)"=w3932) -> ("report out"=w3933:refnum<class "NI_report.lvclass">, "error out"=w3931:errorcluster)  [unwired: 12 in]
                }
                n3117 = local read "TITTLE"() -> (w3879:string)
                n3118 = call-dynamic "Set Report Header Text.vi"("report in"=w3862, "center header text"=w3879, "error in (no error)"=w3861) -> ("report out"=w3900:refnum<class "NI_report.lvclass">, "error out"=w3899:errorcluster)  [unwired: 11 in]
                n3119 = for {
                  N: 1 -> [_]
                  tunnel: [w3938] -> w3886
                  tunnel: [w3937] -> w3885
                  tunnel: w3900 -> [w3936]
                  tunnel: w3899 -> [w3935]
                  n3120 = call-dynamic "New Report Line.vi"("report in"=w3936, "error in (no error)"=w3935) -> ("report out"=w3938:refnum<class "NI_report.lvclass">, "error out"=w3937:errorcluster)  [unwired: 12 in]